vi "UHR-Fleezers Control (host) - 10.8MV_trial2.vi"() -> ()   [LabVIEW 2010] (continued)
        n272 = local read "Location path"() -> (w931:path)
        n273 = Reshape Array(w934, 12) -> (w932:string[])
        n274 = Write to Text File(file (use dialog)=w931, text=w932) -> ()  [unwired: 2 in, 3 out]
      }
      event "Activate Joystick": Value Change {
        n275 = event-data() -> ()  [unwired: 1 in, 5 out]
        n276 = case shown="True" "Activate Joystick" {
          frame False {
          }
          frame True {
            # "Change the trajectory mode to Jog"
            n277 = local read "ESP Port"() -> (w939:refnum<visa-resource-name>)
            n278 = Concatenate Strings("1TJ3;\n2TJ3;\n3TJ3" ("Substring"), "\r") -> (w936:string)
            n279 = VISA Write(VISA resource name=w939, write buffer=w936) -> ()  [unwired: 1 in, 3 out]
          }
        }
      }
    }
  }
  n280 = disable-structure shown="Disabled" {
    disable-tunnel: w24 -> [w968 _]
    frame Disabled {
      w963 = T17 0 items=["Grayscale (U8)", "Grayscale (I16)", "Grayscale (SGL)", "Complex (CSG)", "RGB (U32)", "HSL (U32)", "RGB (U64)", "Grayscale (U16)"] ("Image Type")
      n281 = call <vilib>:"IMAQ Init.vi"("Interface Name"="img0") -> ("error out"=w965:errorcluster, "IMAQ Session Out"=w967:refnum<k11>)  [unwired: 9 in]
      n282 = call <vilib>:"IMAQ Grab Setup.vi"("error in (no error)"=w965, "IMAQ Session In"=w967) -> ("error out"=w961:errorcluster, "IMAQ Session Out"=w962:refnum<k11>)  [unwired: 8 in]
      n283 = call "IMAQ Create"("Image Name"="untitled", "Image Type"=w963) -> ("New Image"=w960:T2)  [unwired: 3 in, 1 out]
      n284 = call <vilib>:"Application Directory.vi"() -> ("Application Directory"=w947:path)
      n285 = Build Path(base path=w947, name or relative path="_trap_screen_positions") -> (appended path=w955:path)
      n286 = Open/Create/Replace File(file path (use dialog)=w955, operation (0:open)=T25."open or create", access (0:read/write)=enum16{"read/write", "read-only", "write-only"}."read/write") -> (refnum out=w957:refnum<file>)  [unwired: 3 in, 2 out]
      n287 = local read "Trap Sets"() -> (w949:u32)
      n288 = for "Load trap positions on video screen from file." {
        N: w949 -> [_]
        tunnel: [w975] -> w950
        tunnel: w957 -> [w974]
        tunnel: [w971] -> w946 mode=indexing
        w973 = 4
        n289 = for {
          N: w973 -> [_]
          tunnel: [w979] -> w975
          tunnel: w974 -> [w978]
          tunnel: w973 -> [w977]
          tunnel: [w976] -> w972 mode=indexing
          n290 = Read from Binary File(5:w977, 11:w978) -> (2:w976:i32, 3:w979:refnum<file>)  [unwired: 4 in, 2 out]
        }
        n291 = Array To Cluster(array=w972) -> (cluster=w971:T29)
      }
      n292 = node-c288() -> (w970:T26)  [unwired: 4 in]
      n293 = timed-loop "acquire video and stage position" {
        timing: w970 -> [_]
        timing-out: [_] -> w969
        tunnel: w962 -> [w998]
        tunnel: w961 -> [w997]
        tunnel: w960 -> [w996]
        tunnel: [w995] -> w942
        tunnel: [w992] -> w943
        tunnel: [w993] -> w941
        tunnel: w968 -> [_]
        shift-right: [w989] -> w959
        shift-left: w946 -> [w990]
        tunnel: w949 -> [w987]
        stop <- w994 stop-if-true
        n294 = node-c288() -> ()  [unwired: 1 in, 1 out]
        n295 = event shown="[2] \"Primary Video Display\": Mouse Down" {
          selector: _ -> [_ _ _ _]
          dyn-events: _ -> [_ _ _ _]
          timeout: 10 -> [_ _ _ _]
          tunnel: w998 -> [w1009 w1024 w1033 w1052]
          tunnel: w997 -> [w1008 w1026 w1031 w1054]
          tunnel: w996 -> [w1007 w1025 w1032 w1053]
          tunnel: [w1006 w1024 w1033 w1052] -> w995
          tunnel: [w999 w1028 FALSE FALSE] -> w994
          tunnel: [w1003 w1026 w1031 w1054] -> w993
          tunnel: [w1002 w1025 w1032 w1053] -> w992
          tunnel: "radius" -> [_ _ w1038 _]
          tunnel: w990 -> [w1000 w1027 w1036 _]
          tunnel: [w1000 w1027 w1037 cluster{i32, i32, i32, i32}[] []] -> w989
          tunnel: w987 -> [_ _ w1029 _]
          event Timeout {
            n296 = event-data() -> ()  [unwired: 1 in, 2 out]
            n297 = call <vilib>:"IMAQ Grab Acquire.vi"("error in (no error)"=w1008, "Image In"=w1007, "IMAQ Session In"=w1009) -> ("error out"=w1004:errorcluster, "Image Out"=w1005:T2, "IMAQ Session Out"=w1006:refnum<k11>)  [unwired: 5 in, 1 out]
            n298 = case shown="True" "trap\nmarkers?" {
              tunnel: w1000 -> [_ w1017]
              tunnel: w1005 -> [w1011 w1016]
              tunnel: w1004 -> [w1010 w1015]
              tunnel: [w1010 w1014] -> w1003
              tunnel: [w1011 w1012] -> w1002
              frame False {
              }
              frame True {
                n299 = for {
                  tunnel: w1017 -> [w1023] mode=indexing
                  shift-right: [w1021] -> w1012
                  shift-left: w1016 -> [w1022]
                  tunnel: w1015 -> [w1020]
                  tunnel: [w1019] -> w1014
                  tunnel: u32 16711680 ("Color") -> [w1018]
                  n300 = call "IMAQ Overlay Oval"("Color"=w1018, "error in (no error)"=w1020, "Bounding Rectangle"=w1023, "Image"=w1022) -> ("error out"=w1019:errorcluster, "Image Out"=w1021:T2)  [unwired: 6 in]
                }
              }
            }
            "Primary Video Display" <- w1002
            n301 = Unbundle By Name(w1004) -> ("status"=w999:bool)
          }
          event "Stop All": Value Change {
            n302 = event-data() -> ()  [unwired: 1 in, 5 out]
            n303 = local read "Stop All"() -> (w1028:bool)
          }
          event "Primary Video Display": Mouse Down {
            n304 = event-data() -> ()  [unwired: 1 in, 7 out]
            n305 = Array Size(array=w1036) -> (size(s)=w1035:i32)
            n306 = Less?(x=w1035, y=w1029) -> (x < y?=w1034:bool)
            n307 = case shown="True" w1034 {
              tunnel: w1038 -> [_ w1048]
              tunnel: w1036 -> [w1039 w1042]
              tunnel: [w1039 w1041] -> w1037
              frame False {
              }
              frame True {
                n308 = property on="Primary Video Display" class="ImageControl"() -> ("Last Mouse Position"=w1040:cluster{"X":i32, "Y":i32})  [unwired: 2 in, 2 out]
                n309 = Unbundle By Name(w1040) -> ("X"=w1050:i32, "Y"=w1049:i32)
                n310 = Add(x=w1049, y=w1048) -> (x+y=w1046:i32)
                n311 = Subtract(x=w1049, y=w1048) -> (x-y=w1044:i32)
                n312 = Add(x=w1050, y=w1048) -> (x+y=w1045:i32)
                n313 = Subtract(x=w1050, y=w1048) -> (x-y=w1047:i32)
                n314 = Bundle(w1047, w1046, w1045, w1044) -> (w1043:cluster{i32, i32, i32, i32})  [unwired: 1 in]
                n315 = Build Array (concatenate)(w1042, w1043) -> (w1041:T30)
              }
            }
          }
          event "clear markers": Value Change {
            n316 = event-data() -> ()  [unwired: 1 in, 5 out]
          }
        }
        n317 = node-c288() -> ()  [unwired: 1 in, 1 out]
      }
      n318 = node-c288(w969) -> ()  [unwired: 1 out]
      n319 = Set File Position(offset (in bytes) (0)=i64 0, refnum=w950, from (0:start)=enum16{"start", "end", "current"}."start") -> (refnum out=w951:refnum<file>)  [unwired: 1 in, 1 out]
      n320 = for "Write trap positions to file so they can be remembered\nwhen program is removed from memory" {
        tunnel: w959 -> [w983] mode=indexing
        tunnel: [w981] -> w958
        tunnel: w951 -> [w980]
        n321 = Cluster To Array(cluster=w983) -> (array=w982:i32[])
        n322 = for {
          tunnel: w982 -> [w986] mode=indexing
          tunnel: [w985] -> w981
          tunnel: w980 -> [w984]
          n323 = Write to Binary File(file (use dialog)=w984, data=w986) -> (refnum out=w985:refnum<file>)  [unwired: 4 in, 2 out]
        }
      }
      n324 = Close File(refnum=w958) -> ()  [unwired: 1 in, 2 out]
      n325 = call "IMAQ Dispose"("Image"=w943, "error in (no error)"=w941) -> ("error out"=w940:errorcluster)  [unwired: 4 in]
      n326 = call <vilib>:"IMAQ Stop.vi"("error in (no error)"=w940, "IMAQ Session In"=w942) -> ("error out"=w944:errorcluster, "IMAQ Session Out"=w945:refnum<k11>)  [unwired: 8 in]
      n327 = call <vilib>:"IMAQ Close.vi"("error in (no error)"=w944, "IMAQ Session In"=w945) -> ()  [unwired: 9 in, 1 out]
    }
    frame Enabled {
    }
  }
  n328 = node-c288(2 ("Processor")) -> (w15:T26)  [unwired: 3 in]
  n329 = node-c288() -> (w69:T26)  [unwired: 4 in]
  n330 = disable-structure shown="Enabled" {
    disable-tunnel: [w1061 _] -> w35
    disable-tunnel: w24 -> [w1060 _]
    frame Enabled {
      n331 = node-c288() -> (w1063:T26)  [unwired: 4 out]
      n332 = timed-loop "Rough control of MCL mirror stage (debugging)" {
        tunnel: w1060 -> [w1066]
        tunnel: [w1065] -> w1061
        timing: w1063 -> [_]
        timing-out: [_] -> w1062
        stop <- w1065 stop-if-true
        n333 = node-c288() -> ()  [unwired: 2 out]
        n334 = case shown="1" "MCL Mode" {
          tunnel: w1066 -> [_ w1069 w1173]
          frame 0, Default {
            # "manual positioning"
          }
          frame 1 {
            # "sinusoidal wave"
            n335 = node-c288() -> (w1071:T26)  [unwired: 4 out]
            n336 = timed-loop "Oscillate MCL mirror" {
              timing: w1071 -> [_]
              timing-out: [_] -> w1070
              tunnel: w1069 -> [w1110]
              i -> [w1109]
              stop <- w1072 stop-if-true
              n337 = node-c288() -> (w1108:i64)  [unwired: 1 out]
              n338 = Multiply(x="AO1", y=32767.0) -> (x*y=w1104:dbl)
              n339 = Multiply(x="AO2", y=32767.0) -> (x*y=w1099:dbl)
              n340 = Divide(x=w1104, y=10.0) -> (x/y=w1105:dbl)
              n341 = Divide(x=w1099, y=10.0) -> (x/y=w1100:dbl)
              n342 = To Word Integer(number=w1105) -> (16bit integer=w1097:i16)
              n343 = To Word Integer(number=w1100) -> (16bit integer=w1096:i16)
              n344 = Divide(x=w1108, y=i64 1000) -> (x/y=w1079:dbl)
              n345 = Multiply(x=w1079, y=w1109) -> (x*y=w1090:dbl)
              n346 = Multiply(x="Osc. freq. (Hz) 2", y=6.283185307179586) -> (x*y=w1091:dbl)
              n347 = Multiply(x=w1091, y=w1090) -> (x*y=w1089:dbl)
              n348 = Sine(x=w1089) -> (sin(x)=w1088:dbl)
              n349 = Multiply(x=w1088, y="Osc. amp. (V)") -> (x*y=w1086:dbl)
              n350 = Add(x=w1086, y="Osc. center (V)") -> (x+y=w1084:dbl)
              n351 = Divide(x=w1084, y=10.0) -> (x/y=w1082:dbl)
              n352 = Multiply(x=w1082, y=32767.0) -> (x*y=w1077:dbl)
              n353 = Select(t=w1077, s="Scan axis", f=w1097) -> (s? t:f=w1095:dbl)
              n354 = Select(t=w1096, s="Scan axis", f=w1077) -> (s? t:f=w1094:dbl)
              n355 = local read "MCL Mode"() -> (w1076:u16)
              n356 = Not Equal?(x=w1076, y=u16 1) -> (x != y?=w1073:bool)
              n357 = local read "Stop All"() -> (w1074:bool)
              n358 = xnode "Read/Write Control"("FPGA VI Reference In"=w1110, "AO1"=w1095, "AO2"=w1094) -> ()  [unwired: 1 in, 2 out]
              n359 = Compound Arithmetic op=OR(w1074, w1073) -> (w1072:bool)
              n360 = node-c288() -> ()  [unwired: 2 out]
            }
            n361 = node-c288(w1070) -> ()  [unwired: 1 out]
          }
          frame 2 {
            # "linear scan"
            n362 = case shown="True" "Start Scan" {
              tunnel: w1173 -> [_ w1185]
              frame False {
              }
              frame True {
                n363 = Subtract(x="End (V)", y="Begin (V)") -> (x-y=w1181:dbl)
                n364 = Decrement(x="N Points") -> (x-1=w1180:dbl)
                n365 = Divide(x=w1181, y=w1180) -> (x/y=w1178:dbl)
                n366 = for {
                  N: "N Points" -> [_]
                  tunnel: "Begin (V)" -> [w1198]
                  tunnel: w1185 -> [w1190]
                  tunnel: [w1189] -> w1184 mode=indexing
                  tunnel: w1178 -> [w1188]
                  tunnel: [w1186] -> w1177 mode=indexing
                  i -> [w1197]
                  n367 = Multiply(x=w1188, y=w1197) -> (x*y=w1196:dbl)
                  n368 = Add(x=w1198, y=w1196) -> (x+y=w1193:dbl)
                  n369 = local read "Scan axis"() -> (w1187:bool)
                  n370 = local read "AO1"() -> (w1195:dbl)
                  n371 = local read "AO2"() -> (w1194:dbl)
                  n372 = Select(t=w1193, s=w1187, f=w1195) -> (s? t:f=w1192:dbl)
                  n373 = Select(t=w1194, s=w1187, f=w1193) -> (s? t:f=w1191:dbl)
                  n374 = flat-sequence {
                    tunnel: w1192 -> [w1202]
                    tunnel: w1191 -> [w1201]
                    tunnel: w1190 -> [w1199]
                    tunnel: [w1269] -> w1189
                    tunnel: [w1268] -> w1186
                    frame #0 {
                      w1205 = 10.0 ("y")
                      w1200 = 32767.0 ("y")
                      n375 = Multiply(x=w1202, y=w1200) -> (x*y=w1208:dbl)
                      n376 = Multiply(x=w1201, y=w1200) -> (x*y=w1206:dbl)
                      n377 = Divide(x=w1208, y=w1205) -> (x/y=w1209:dbl)
                      n378 = Divide(x=w1206, y=w1205) -> (x/y=w1207:dbl)
                      n379 = To Word Integer(number=w1209) -> (16bit integer=w1203:i16)
                      n380 = To Word Integer(number=w1207) -> (16bit integer=w1204:i16)
                      n381 = xnode "Read/Write Control"("FPGA VI Reference In"=w1199, "AO1"=w1203, "AO2"=w1204) -> ()  [unwired: 1 in, 2 out]
                    }
                    frame #1 {
                      n382 = Wait (ms)(milliseconds to wait="DAQ Delay (ms)") -> ()  [unwired: 1 out]
                    }
                    frame #2 {
                      n383 = local read "Slow mean"() -> (w1269:dbl)
                      n384 = local read "Sigma"() -> (w1268:dbl)
                    }
                  }
                }
                n385 = Bundle("Begin (V)"="Begin (V)", w1178, w1184) -> (→"MCL Scan":cluster{"Begin (V)":dbl, dbl, dbl[]})  [unwired: 1 out]
                n386 = Bundle("Begin (V)"="Begin (V)", w1178, w1177) -> (→"MCL Scan 2":cluster{"Begin (V)":dbl, dbl, dbl[]})  [unwired: 1 out]
              }
            }
          }
        }
        n387 = local read "Stop All"() -> (w1065:bool)
        n388 = node-c288() -> ()  [unwired: 2 out]
      }
      n389 = node-c288(w1062) -> ()  [unwired: 1 out]
    }
    frame Disabled {
    }
  }
  n390 = timed-loop "Control parameters (event loop)" {
    tunnel: w24 -> [w1275]
    shift-right: [w1274] -> _
    shift-left: errorcluster {"status"=FALSE, "code"=0, "source"=""} ("error out") -> [w1273]
    tunnel: [w1272] -> w37
    timing: w15 -> [_]
    timing-out: [_] -> w14
    stop <- w1272 stop-if-true
    n391 = node-c288() -> ()  [unwired: 1 in, 1 out]
    n392 = event shown="[6] \"BD 1 Frequency 1 (MHz)\", \"BD 1 Frequency 2 (MHz)\", \"BD 1 Frequency 3 (MHz)\", \"BD 2 Frequency 1 (MHz)\", \"BD 2 Frequency 2 (MHz)\", \"BD 2 Frequency 3 (MHz)\", \"Trap Delta (MHz)\": Value Change" {
      selector: _ -> [_ _ _ _ _ _ _ _ _ _ _ _ _ _ _ _ _ _ _ _ _ _ _ _ _ _ _ _ _ _ _ _ _ _ _ _ _ _ _ _ _ _ _ _ _ _ _ _ _ _ _ _ _ _ _]
      dyn-events: _ -> [_ _ _ _ _ _ _ _ _ _ _ _ _ _ _ _ _ _ _ _ _ _ _ _ _ _ _ _ _ _ _ _ _ _ _ _ _ _ _ _ _ _ _ _ _ _ _ _ _ _ _ _ _ _ _]
      timeout: _ -> [_ _ _ _ _ _ _ _ _ _ _ _ _ _ _ _ _ _ _ _ _ _ _ _ _ _ _ _ _ _ _ _ _ _ _ _ _ _ _ _ _ _ _ _ _ _ _ _ _ _ _ _ _ _ _]
      tunnel: w1275 -> [w1313 _ _ _ w1435 _ w1532 _ w1596 _ _ _ w1791 _ _ w1893 w2037 w2101 w2176 w2330 w2407 w2538 w2634 w2720 w2806 w2892 w2978 w3064 w3157 w3321 w3532 _ w3677 w3814 _ w4021 w4063 w4111 w4190 w4232 _ w4278 _ _ _ _ w4469 _ w4562 w4603 w4650 w4838 w4887 _ w4949]
      tunnel: [w1312 _ _ _ w1425 _ w1531 _ w1559 _ w1756 _ w1770 _ _ w1892 w2033 w2098 w2173 w2329 w2405 w2537 w2628 w2714 w2800 w2886 w2972 w3058 w3155 w3320 w3530 _ w3675 w3812 _ w4019 w4061 w4101 w4188 w4230 _ w4276 _ _ _ _ w4467 _ _ _ _ _ _ _ _] -> w1274
      tunnel: w1273 -> [w1311 _ _ _ w1434 _ w1530 _ w1591 _ w1756 _ w1790 _ _ w1891 w2032 w2097 w2172 w2328 w2406 w2536 w2633 w2719 w2805 w2891 w2977 w3063 w3156 w3319 w3531 _ w3676 w3813 _ w4020 w4062 w4110 w4189 w4231 _ w4277 _ _ _ _ w4468 _ w4561 w4602 w4649 w4837 w4886 _ w4948]
      tunnel: [_ _ _ _ _ _ _ _ _ _ w1755 _ _ _ _ _ _ _ _ _ _ _ _ _ _ _ _ _ _ _ _ _ _ _ _ _ _ _ _ _ _ _ _ _ _ _ _ _ _ _ _ _ _ _ _] -> w1272
      tunnel: [_ _ _ _ _ _ _ "Round T1 X" _ _ _ _ _ _ _ _ _ _ _ _ _ _ _ _ _ _ _ _ _ _ _ _ _ _ _ _ _ _ _ _ _ _ _ _ _ _ _ _ _ _ _ _ _ _ _] -> _
      tunnel: [_ _ _ "Adjust Scale\nto Mean" _ _ _ _ _ _ _ _ _ _ _ _ _ _ _ _ _ _ _ _ _ _ _ _ _ _ _ _ _ _ _ _ _ _ _ _ _ _ _ _ _ _ _ _ _ _ _ _ "Set SP to Reading" _ _] -> _
      tunnel: [_ _ _ _ _ _ _ _ _ "Round T2 X" _ "Delayed Interlace Start" _ _ _ _ _ _ _ _ _ _ _ _ _ _ _ _ _ _ _ _ _ _ _ _ _ _ _ _ _ _ _ _ _ _ _ _ _ _ _ _ _ _ _] -> _
      event "AI Count (ticks)", "Sets to FIFO (Traps)", "Save ave N", "FPGA Ave.", "# Samples/channel", "N sets to save": Value Change {
        # "So that if 'Save ave N' is updated, the AOD scanning code updates too."
        n393 = event-data() -> ()  [unwired: 6 out]
        n394 = local read "AI Count (ticks)"() -> (w1293:u32)
        n395 = Boolean To (0,1)(Boolean="Sets to FIFO (Traps)") -> (0, 1=w1303:cluster{"Set 1":i16, "Set 2":i16, "Set 3":i16})
        n396 = xnode "Read/Write Control"("FPGA VI Reference In"=w1313, "error in"=w1311, "ai count"=w1293, "AI1 Sets to FIFO"="Sets to FIFO (Traps)", "N of AI1 Int Acq Sets"="N Acq Sets (Traps + Fl.)") -> ("error out"=w1312:errorcluster)  [unwired: 1 out]
        n397 = Cluster To Array(cluster=w1303) -> (array=w1302:i16[])
        n398 = To Unsigned Long Integer(number=w1302) -> (unsigned 32bit integer=w1282:u32[])
        n399 = local read "Scan steps (AOD)"() -> (w1304:u64)
        n400 = Multiply(x=w1293, y="N Acq Sets (Traps + Fl.)") -> (x*y=w1291:u32)
        n401 = Divide(x=40000000.0, y=w1293) -> (x/y=w1285:dbl)
        "AI rate (Hz)" <- w1285
        "Ave. Rate (Hz)" <- w1285
        n402 = Add Array Elements(numeric array=w1282) -> (sum=w1294:u32)
        "Trap Sets" <- w1294
        n403 = Reciprocal(x=w1285) -> (1/x=→"Ave. Period (s)":dbl)
        n404 = property on="Scan steps (AOD)" class="DigNum (strict)"("Val(Sgnl)"=w1304) -> ()  [unwired: 2 in, 2 out]
        n405 = Divide(x=w1285, y="N Acq Sets (Traps + Fl.)") -> (x/y=w1308:dbl)
        "Data Rate (Hz)" <- w1308
        n406 = Reciprocal(x=w1308) -> (1/x=→"Data Period (s)":dbl)
        n407 = local read "Save ave N"() -> (w1307:dbl)
        n408 = Divide(x=w1308, y=w1307) -> (x/y=w1306:dbl)
        "Save Data Rate (Hz)" <- w1306
        n409 = Reciprocal(x=w1306) -> (1/x=→"Save Data Period (s)":dbl)
        n410 = Multiply(x=w1291, y="# Samples/trap") -> (x*y=w1289:u32)
        "Counts/DMA" <- w1289
        n411 = property on="Trap Disp. Downsample" class="DigNum (strict)"("Maximum"="# Samples/trap") -> ()  [unwired: 2 in, 2 out]
        n412 = Multiply(x=w1294, y="# Samples/trap") -> (x*y=w1283:u32)
        "# Samples/channel" <- w1283
        n413 = Multiply(x=w1283, y=u32 8) -> (x*y=→"Trap AI Elements/DMA read":u32)
        n414 = local read "APD Int. Count"() -> (w1290:u32)
        n415 = Multiply(x=w1283, y=u32 3) -> (x*y=→"Trap Pos Elements/DMA read":u32)
        n416 = Divide(x=w1289, y=w1290) -> (x/y=w1280:dbl)
        "APD Samples/FIFO Acq." <- w1280
        n417 = Divide(x=w1289, y=40000000.0) -> (x/y=w1287:dbl)
        "DMA Update Period (s)" <- w1287
        n418 = Multiply(x=2.0, y=w1280) -> (x*y=→"APD Elements/DMA read":dbl)
        n419 = property on="APD Disp. Downsample" class="DigNum (strict)"("Maximum"=w1280) -> ()  [unwired: 2 in, 2 out]
        n420 = local read "N sets to save"() -> (w1300:u32)
        n421 = Multiply(x=w1287, y=w1300) -> (x*y=→"Total Time (s)":dbl)
        "FPGA Averaging" <- FALSE ("FPGA Averaging")
      }
      event "Rescale on Mean": Value Change {
        n422 = event-data() -> ()  [unwired: 7 out]
        n423 = And(x=FALSE, y="Rescale on Mean") -> (x .and. y?=w1400:bool)
        n424 = local write "Rescale on Mean"(w1400) -> ()
        n425 = local read "Bead Mean (nm)"() -> (w1405:dbl)
        n426 = Add(x="Amplitude (nm)", y=w1405) -> (x+y=w1403:dbl)
        n427 = Subtract(x=w1405, y="Amplitude (nm)") -> (x-y=w1402:dbl)
        n428 = property on="Bead Separation" class="WFChart (strict)"("YScale.Minimum"=w1402) -> ()  [unwired: 2 in, 2 out]
        n429 = property on="Bead Separation" class="WFChart (strict)"("YScale.Maximum"=w1403) -> ()  [unwired: 2 in, 2 out]
      }
      event "Detector Type": Value Change {
        n430 = event-data() -> ()  [unwired: 7 out]
        n431 = local read "AI labels"() -> (w1406:string[])
        n432 = property on="High Res. Display" class="Ring (strict)"("Strings []"=w1406) -> ()  [unwired: 2 in, 2 out]
        n433 = Build Array (concatenate)(w1406, "none") -> (w1407:string[])
        n434 = property on="FFT 1 Choice 1" class="Ring (strict)"("Strings []"=w1407) -> ()  [unwired: 2 in, 2 out]
        n435 = property on="FFT 1 Choice 2" class="Ring (strict)"("Strings []"=w1407) -> ()  [unwired: 2 in, 2 out]
        n436 = property on="FFT 2 Choice 1" class="Ring (strict)"("Strings []"=w1407) -> ()  [unwired: 2 in, 2 out]
        n437 = property on="FFT 2 Choice 2" class="Ring (strict)"("Strings []"=w1407) -> ()  [unwired: 2 in, 2 out]
        n438 = Bundle("APD 1", "APD 2") -> (w1410:cluster{string, string})  [unwired: 1 out]
        n439 = Cluster To Array(cluster=w1410) -> (array=w1408:string[])
        n440 = Build Array (concatenate)(w1408, w1407) -> (w1412:string[])
        n441 = Array Size(array=w1412) -> (size(s)=w1413:i32)
        n442 = property on="Signals to Plot" class="LstBox (strict)"("Item Names"=w1412) -> ()  [unwired: 2 in, 2 out]
        n443 = property on="Signals to Plot" class="LstBox (strict)"("Number of Rows"=w1413) -> ()  [unwired: 2 in, 2 out]
        n444 = property on="All Signals" class="WFChart (strict)"("LegNumRows"=w1413) -> ()  [unwired: 2 in, 2 out]
      }
      event "Adjust Scale\nto Mean": Value Change {
        n445 = event-data() -> ()  [unwired: 7 out]
        n446 = local read "APD 1 Rate (Hz)"() -> (w1422:dbl)
        n447 = Multiply(x=1000.0, y="Above (kHz)") -> (x*y=w1420:dbl)
        n448 = Multiply(x=1000.0, y="Below (kHz)") -> (x*y=w1418:dbl)
        n449 = Add(x=w1420, y=w1422) -> (x+y=w1415:dbl)
        n450 = Subtract(x=w1422, y=w1418) -> (x-y=w1416:dbl)
        n451 = property on="APD Chart" class="WFChart (strict)"("YScale.Minimum"=w1416) -> ()  [unwired: 2 in, 2 out]
        n452 = property on="APD Chart" class="WFChart (strict)"("YScale.Maximum"=w1415) -> ()  [unwired: 2 in, 2 out]
      }
      event "Phase adj. (AI1)", "+ phase (AI1)", "- phase (AI1)": Value Change {
        n453 = event-data() -> ()  [unwired: 7 out]
        n454 = Negate(x="Phase adj. (AI1)") -> (-x=w1432:i16)
        n455 = Select(t=w1432, s="- phase (AI1)", f="Phase adj. (AI1)") -> (s? t:f=w1431:i16)
        n456 = xnode "Read/Write Control"("FPGA VI Reference In"=w1435, "error in"=w1434, "Phase count adjustment"=w1431) -> ("FPGA VI Reference Out"=w1430:T19, "error out"=w1429:errorcluster)
        n457 = Or(x="- phase (AI1)", y="+ phase (AI1)") -> (x .or. y?=w1426:bool)
        n458 = xnode "Read/Write Control"("FPGA VI Reference In"=w1430, "error in"=w1429, "+ phase"=w1426) -> ("error out"=w1425:errorcluster)  [unwired: 1 out]
      }
      event "Signals to Plot": Double Click {
        w1513 = u32 9868950 ("Color Box")
        n459 = event-data() -> ("Row"=w1515:i32)  [unwired: 9 out]
        n460 = property on="All Signals" class="WFChart (strict)"("Active Plot"=w1515) -> (error out=w1526:errorcluster)  [unwired: 2 in, 1 out]
        n461 = property on="All Signals" class="WFChart (strict)" props=["Plot", "Visible?", "Plot", "Plot Color"](error in=w1526) -> (error out=w1525:errorcluster, "Plot.Visible?"=w1524:bool)  [unwired: 1 in, 2 out]
        n462 = Select(t=FALSE ("Plot.Visible"), s=w1524, f=TRUE ("Plot.Visible")) -> (s? t:f=w1519:bool)
        n463 = property on="All Signals" class="WFChart (strict)"(error in=w1525, "Plot.Visible?"=w1519) -> (error out=w1521:errorcluster)  [unwired: 1 in, 1 out]
        n464 = property on="All Signals" class="WFChart (strict)"(error in=w1521) -> (error out=w1516:errorcluster, "Plot.Plot Color"=w1520:u32)  [unwired: 1 in, 1 out]
        n465 = property on="Signals to Plot" class="LstBox (strict)"(error in=w1516, "Active Row"=w1515) -> (error out=w1514:errorcluster)  [unwired: 1 in, 1 out]
        n466 = Select(t=w1520, s=w1519, f=u32 0) -> (s? t:f=w1517:u32)
        n467 = property on="Signals to Plot" class="LstBox (strict)"(error in=w1514, "CellFontColor"=w1517, "SelColor"=w1513, "CellBG"=w1513, "CellFontSize"=u32 20 ("Active Row:Cell Font:Size"), "CellFontBold"=TRUE ("Active Row:Cell Font:Bold")) -> ()  [unwired: 1 in, 2 out]
      }
      event "BD 1 Frequency 1 (MHz)", "BD 1 Frequency 2 (MHz)", "BD 1 Frequency 3 (MHz)", "BD 2 Frequency 1 (MHz)", "BD 2 Frequency 2 (MHz)", "BD 2 Frequency 3 (MHz)", "Trap Delta (MHz)": Value Change {
        # "anytime one of the frequencies is changed, write it to the RF board UNLESS Set 2 is being oscillated. The oscillation\nscript writes the frequencies to the RF board."
        n468 = event-data() -> ("CtlRef"=w1529:refnum<vi>)  [unwired: 6 out]
        n469 = control-ref of="Trap Delta (MHz)"() -> (w1528:refnum<vi>)
        n470 = Equal?(x=w1528, y=w1529) -> (x = y?=w1527:bool)
        n471 = case shown="False" "Oscillate Set 2" {
          tunnel: w1532 -> [w1552 _]
          tunnel: [w1551 w1555] -> w1531
          tunnel: w1530 -> [w1550 w1555]
          tunnel: w1527 -> [w1536 _]
          frame False {
            n472 = local read "BD 1 Frequency 1 (MHz)"() -> (w1534:dbl)
            n473 = local read "BD 1 Frequency 2 (MHz)"() -> (w1538:dbl)
            n474 = Add(x=w1534, y="Trap Delta (MHz)") -> (x+y=w1537:dbl)
            n475 = Select(t=w1537, s=w1536, f=w1538) -> (s? t:f=w1535:dbl)
            n476 = local read "Y RF Frequency Limits (MHz)"() -> (w1540:T16)
            n477 = local read "X RF Frequency Limits (MHz)"() -> (w1541:T16)
            n478 = local read "BD 1 Frequency 3 (MHz)"() -> (w1553:dbl)
            n479 = local write "BD 1 Frequency 2 (MHz)"(w1535) -> ()
            n480 = local read "BD 2 Frequency 1 (MHz)"() -> (w1544:dbl)
            n481 = local read "BD 2 Frequency 2 (MHz)"() -> (w1543:dbl)
            n482 = local read "BD 2 Frequency 3 (MHz)"() -> (w1554:dbl)
            n483 = call "set RF board frequency - interlace.vi"("Board 2 Frequency Limits"=w1540, "Board 1 Frequency Limits"=w1541, "error in"=w1550, "FPGA VI Reference In"=w1552, "Board 2 Frequency 3 (MHz)"=w1554, "Board 1 Frequency 3 (MHz)"=w1553, "Board 2 Frequency 2 (MHz)"=w1543, "Board 2 Frequency 1 (MHz)"=w1544, "Board 1 Frequency 2 (MHz)"=w1535, "Board 1 Frequency 1  (MHz)"=w1534) -> ("error out"=w1551:errorcluster)  [unwired: 1 out]
            n484 = Subtract(x=w1544, y=w1543) -> (x-y=w1548:dbl)
            n485 = Subtract(x=w1535, y=w1534) -> (x-y=w1549:dbl)
            n486 = Square(x=w1548) -> (x^2=w1546:dbl)
            n487 = Square(x=w1549) -> (x^2=w1547:dbl)
            n488 = Add(x=w1547, y=w1546) -> (x+y=w1545:dbl)
            n489 = Square Root(x=w1545) -> (sqrt(x)=w1542:dbl)
            n490 = local write "Trap Delta (MHz)"(w1542) -> ()
            n491 = property on="Initial delta (MHz)" class="DigNum (strict)"("Val(Sgnl)"=w1542) -> ()  [unwired: 2 in, 2 out]
          }
          frame True {
          }
        }
      }
      event "Round T1 X": Value Change {
        n492 = event-data() -> ()  [unwired: 7 out]
        n493 = local read "BD 1 Frequency 1 (MHz)"() -> (w1558:dbl)
        n494 = Round To Nearest(number=w1558) -> (nearest integer value=w1557:dbl)
        n495 = property on="BD 1 Frequency 1 (MHz)" class="DigNum (strict)"("Val(Sgnl)"=w1557) -> ()  [unwired: 2 in, 2 out]
      }
      event "Restart RF": Value Change {
        n496 = event-data() -> ()  [unwired: 7 out]
        n497 = xnode "Read/Write Control"("FPGA VI Reference In"=w1596, "error in"=w1591, "FPGA Controls  RF Box"=FALSE) -> ("FPGA VI Reference Out"=w1595:T19, "error out"=w1590:errorcluster)
        n498 = local read "Y RF Amplitude Limits (%)"() -> (w1571:T16)
        n499 = local read "X RF Amplitude Limits (%)"() -> (w1572:T16)
        n500 = local read "X RF Frequency Limits (MHz)"() -> (w1574:T16)
        n501 = local read "Y RF Frequency Limits (MHz)"() -> (w1573:T16)
        n502 = xnode "Read/Write Control"("FPGA VI Reference In"=w1595, "error in"=w1590, "Direct RF Box  Communication"=TRUE) -> ("FPGA VI Reference Out"=w1594:T19, "error out"=w1589:errorcluster)
        n503 = local read "BD 2 Frequency 3 (MHz)"() -> (w1581:dbl)
        n504 = local read "BD 2 Frequency 2 (MHz)"() -> (w1582:dbl)
        n505 = local read "BD 1 Frequency 3 (MHz)"() -> (w1585:dbl)
        n506 = local read "BD 1 Frequency 1 (MHz)"() -> (w1586:dbl)
        n507 = local read "BD 2 Frequency 1 (MHz)"() -> (w1583:dbl)
        n508 = local read "BD 1 Frequency 2 (MHz)"() -> (w1584:dbl)
        n509 = call "Initialize RF boards - interlace 3.vi"("error in"=w1589, "FPGA VI Reference In"=w1594) -> ("error out"=w1588:errorcluster, "FPGA VI Reference Out"=w1593:T19)
        n510 = local read "BD 2 Amplitude 2 (%)"() -> (w1576:dbl)
        n511 = local read "BD 2 Amplitude 1 (%)"() -> (w1577:dbl)
        n512 = local read "BD 2 Amplitude 3 (%)"() -> (w1575:dbl)
        n513 = local read "BD 1 Amplitude 3 (%)"() -> (w1580:dbl)
        n514 = local read "BD 1 Amplitude 1 (%)"() -> (w1579:dbl)
        n515 = local read "BD 1 Amplitude 2 (%)"() -> (w1578:dbl)
        n516 = call "set RF board frequency - interlace.vi"("Board 2 Frequency Limits"=w1573, "Board 1 Frequency Limits"=w1574, "error in"=w1588, "FPGA VI Reference In"=w1593, "Board 2 Frequency 3 (MHz)"=w1581, "Board 1 Frequency 3 (MHz)"=w1585, "Board 2 Frequency 2 (MHz)"=w1582, "Board 2 Frequency 1 (MHz)"=w1583, "Board 1 Frequency 2 (MHz)"=w1584, "Board 1 Frequency 1  (MHz)"=w1586) -> ("error out"=w1587:errorcluster, "FPGA VI Reference Out"=w1592:T19)
        n517 = call "set RF board amplitude - interlace.vi"("Board 2 Amplitude Limits"=w1571, "Board 1 Amplitude Limits"=w1572, "error in"=w1587, "FPGA VI Reference In"=w1592, "Board 2 Amplitude 3 (%)"=w1575, "Board 1 Amplitude 3 (%)"=w1580, "Board 2 Amplitude 2 (%)"=w1576, "Board 2 Amplitude 1 (%)"=w1577, "Board 1 Amplitude 2 (%)"=w1578, "Board 1 Amplitude 1 (%)"=w1579) -> ("error out"=w1564:errorcluster, "FPGA VI Reference Out"=w1568:T19)
        n518 = xnode "Read/Write Control"("FPGA VI Reference In"=w1568, "error in"=w1564, "Direct RF Box  Communication"=FALSE) -> ("FPGA VI Reference Out"=w1567:T19, "error out"=w1566:errorcluster)
        n519 = flat-sequence {
          tunnel: w1566 -> [w1597]
          tunnel: [w1597] -> w1565
          frame #0 {
            n520 = Wait (ms)(milliseconds to wait=u32 50) -> ()  [unwired: 1 out]
          }
        }
        n521 = xnode "Read/Write Control"("FPGA VI Reference In"=w1567, "error in"=w1565, "FPGA Controls  RF Box"=TRUE) -> ("error out"=w1560:errorcluster)  [unwired: 1 out]
        n522 = property on="Restart RF" class="Bool (strict)"(error in=w1560, "Value"=FALSE ("Restart RF")) -> (error out=w1559:errorcluster)  [unwired: 1 in, 1 out]
      }
      event "Round T2 X": Value Change {
        n523 = event-data() -> ()  [unwired: 7 out]
        n524 = local read "BD 1 Frequency 2 (MHz)"() -> (w1752:dbl)
        n525 = Round To Nearest(number=w1752) -> (nearest integer value=w1751:dbl)
        n526 = property on="BD 1 Frequency 2 (MHz)" class="DigNum (strict)"("Val(Sgnl)"=w1751) -> ()  [unwired: 2 in, 2 out]
      }
      event "Stop All": Value Change {
        n527 = event-data() -> ()  [unwired: 7 out]
        n528 = call "hamilton_controller.vi"("action"=T22."DISCONNECT") -> ()  [unwired: 10 in, 1 out]
        n529 = local read "Stop All"() -> (w1755:bool)
      }
      event "Delayed Interlace Start": Value Change {
        n530 = event-data() -> ()  [unwired: 7 out]
        n531 = flat-sequence {
          frame #0 {
            n532 = Multiply(x="Delay to Interlace (s)", y=1000.0) -> (x*y=w1758:dbl)
            n533 = Wait (ms)(milliseconds to wait=w1758) -> ()  [unwired: 1 out]
          }
          frame #1 {
            n534 = property on="Green laser mode" class="RadioBtnsControl (strict)"("Val(Sgnl)"=enum32{"Laser ON", "Laser OFF", "Interlace"}."Interlace" ("Value (Signaling)")) -> ()  [unwired: 2 in, 2 out]
          }
        }
      }
      event "BD 1 Amplitude 1 (%)", "BD 1 Amplitude 2 (%)", "BD 1 Amplitude 3 (%)", "BD 2 Amplitude 1 (%)", "BD 2 Amplitude 2 (%)", "BD 2 Amplitude 3 (%)", "Trap 1 ON", "Trap 2 ON", "Trap 3 ON", "Feedback On/Off", "All FB On/Off": Value Change {
        w1782 = i16 1 ("f")
        n535 = event-data() -> ()  [unwired: 7 out]
        n536 = local write "Trap 1 (ON/OFF)"("Trap 1 ON") -> ()
        n537 = local write "Trap 2 (ON/OFF)"("Trap 2 ON") -> ()
        n538 = Boolean To (0,1)(Boolean="Trap 3 ON") -> (0, 1=w1783:i16)
        n539 = Boolean To (0,1)(Boolean="Trap 1 ON") -> (0, 1=w1784:i16)
        n540 = Boolean To (0,1)(Boolean="Trap 2 ON") -> (0, 1=w1785:i16)
        n541 = Select(t=w1785, s="Trap ON/OFF X or Y Amp?", f=w1782) -> (s? t:f=w1780:i16)
        n542 = Select(t=w1784, s="Trap ON/OFF X or Y Amp?", f=w1782) -> (s? t:f=w1781:i16)
        n543 = Select(t=w1783, s="Trap ON/OFF X or Y Amp?", f=w1782) -> (s? t:f=w1779:i16)
        n544 = Select(t=w1782, s="Trap ON/OFF X or Y Amp?", f=w1785) -> (s? t:f=w1777:i16)
        n545 = Select(t=w1782, s="Trap ON/OFF X or Y Amp?", f=w1784) -> (s? t:f=w1778:i16)
        n546 = Select(t=w1782, s="Trap ON/OFF X or Y Amp?", f=w1783) -> (s? t:f=w1776:i16)
        n547 = And(x="All FB On/Off", y="Feedback On/Off") -> (x .and. y?=w1774:cluster{"Set 1":bool, "Set 2":bool})
        n548 = local read "BD 1 Amplitude 1 (%)"() -> (w1794:dbl)
        n549 = local read "BD 1 Amplitude 2 (%)"() -> (w1793:dbl)
        n550 = local read "BD 1 Amplitude 3 (%)"() -> (w1792:dbl)
        n551 = Unbundle By Name(w1774) -> ("Set 1"=w1769:bool, "Set 2"=w1766:bool)
        n552 = local read "Y RF Amplitude Limits (%)"() -> (w1762:T16)
        n553 = local read "X RF Amplitude Limits (%)"() -> (w1763:T16)
        n554 = local read "BD 2 Amplitude 1 (%)"() -> (w1795:dbl)
        n555 = local read "BD 2 Amplitude 2 (%)"() -> (w1796:dbl)
        n556 = local read "BD 2 Amplitude 3 (%)"() -> (w1797:dbl)
        n557 = And(x="Trap 2 ON", y=w1766) -> (x .and. y?=w1764:bool)
        n558 = And(x="Trap 1 ON", y=w1769) -> (x .and. y?=w1767:bool)
        n559 = Multiply(x=w1781, y=w1794) -> (x*y=w1789:dbl)
        n560 = Multiply(x=w1793, y=w1780) -> (x*y=w1787:dbl)
        n561 = Multiply(x=w1792, y=w1779) -> (x*y=w1788:dbl)
        n562 = Multiply(x=w1795, y=w1778) -> (x*y=w1798:dbl)
        n563 = Multiply(x=w1796, y=w1777) -> (x*y=w1799:dbl)
        n564 = Multiply(x=w1797, y=w1776) -> (x*y=w1800:dbl)
        n565 = call "set RF board amplitude - interlace.vi"("Board 2 Amplitude Limits"=w1762, "Board 1 Amplitude Limits"=w1763, "error in"=w1790, "FPGA VI Reference In"=w1791, "Board 2 Amplitude 3 (%)"=w1800, "Board 1 Amplitude 3 (%)"=w1788, "Board 2 Amplitude 2 (%)"=w1799, "Board 2 Amplitude 1 (%)"=w1798, "Board 1 Amplitude 2 (%)"=w1787, "Board 1 Amplitude 1 (%)"=w1789) -> ("error out"=w1771:errorcluster, "FPGA VI Reference Out"=w1772:T19)
        n566 = xnode "Read/Write Control"("FPGA VI Reference In"=w1772, "error in"=w1771, "FB On/Off Set 1"=w1767, "FB On/Off Set 2"=w1764) -> ("error out"=w1770:errorcluster)  [unwired: 1 out]
      }
      event "Load parameters": Value Change {
        n567 = event-data() -> ()  [unwired: 7 out]
        n568 = property on="Saved AOD Raster Scan Parameter Sets" class="Arr (strict)"() -> ("Index Values"=w1870:u32[])  [unwired: 2 in, 2 out]
        n569 = Index Array(array=w1870, index=0) -> (element=w1867:u32)
        n570 = local write "Load parameters"(FALSE ("Load parameters")) -> ()
        n571 = Index Array(array="Saved AOD Raster Scan Parameter Sets", index=w1867) -> (element=w1866:T32)
        n572 = Unbundle By Name(w1866) -> ("Scan Range AOD (nm) 2"=w1865:dbl, "Step Size AOD (nm) 2"=w1864:dbl, "Scan Speed AOD (nm/s) 2"=w1863:dbl, "Number of scans (AOD) 2"=w1862:u16)
        n573 = flat-sequence {
          tunnel: w1865 -> [w1873]
          tunnel: w1864 -> [w1872]
          tunnel: w1863 -> [w1871]
          tunnel: w1862 -> [w1874]
          frame #0 {
            n574 = local write "Scan Speed (nm/s)"(w1871) -> ()
            n575 = local write "Scan Range (nm)"(w1873) -> ()
            n576 = local write "Step Size (nm)"(w1872) -> ()
          }
          frame #1 {
            n577 = property on="Number of F/B Scans (AOD)" class="DigNum (strict)"("Val(Sgnl)"=w1874) -> ()  [unwired: 2 in, 2 out]
          }
        }
      }
      event "Trap 1 (ON/OFF)", "Trap 2 (ON/OFF)": Value Change {
        n578 = event-data() -> ()  [unwired: 7 out]
        n579 = property on="Trap 2 ON" class="Bool (strict)"("Val(Sgnl)"="Trap 2 (ON/OFF)") -> ()  [unwired: 2 in, 2 out]
        n580 = property on="Trap 1 ON" class="Bool (strict)"("Val(Sgnl)"="Trap 1 (ON/OFF)") -> ()  [unwired: 2 in, 2 out]
      }
      event "DIO count 1 (ticks)", "DIO count 2 (ticks)", "DIO count 3 (ticks)", "Interlace", "Number Interlace Sets", "Not-Interlacing Set": Value Change {
        n581 = event-data() -> ()  [unwired: 7 out]
        n582 = local read "DIO count 3 (ticks)"() -> (w1887:u32)
        n583 = local read "DIO count 1 (ticks)"() -> (w1889:u32)
        n584 = local read "DIO count 2 (ticks)"() -> (w1888:u32)
        n585 = To Unsigned Byte Integer(number="Not-Interlacing Set") -> (unsigned 8bit integer=w1878:u8)
        n586 = Add(x=w1878, y=u8 1) -> (x+y=w1882:u8)
        n587 = xnode "Read/Write Control"("FPGA VI Reference In"=w1893, "error in"=w1891, "DIO count 1 (ticks)"=w1889, "DIO count 2 (ticks)"=w1888, "DIO count 3 (ticks)"=w1887, "Interlace ON/OFF"="Interlace", "Number Interlace Cycles"="Number Interlace Sets", "Interlace Off Parameters"=w1882) -> ("error out"=w1892:errorcluster)  [unwired: 1 out]
        n588 = Build Array(w1889, w1888, w1887) -> (w1880:u32[])
        n589 = Split 1D Array(array=w1880, index="Number Interlace Sets") -> (first subarray=w1890:u32[])  [unwired: 1 out]
        n590 = Index Array(array=w1880, index=w1878) -> (element=w1879:u32)
        n591 = Add Array Elements(numeric array=w1890) -> (sum=w1884:u32)
        n592 = Select(t=w1884, s="Interlace", f=w1879) -> (s? t:f=→"Total Counts (ticks)":u32)
      }
      event "Reset Feedback": Value Change {
        n593 = event-data() -> ()  [unwired: 7 out]
        n594 = Unbundle By Name("Reset Feedback") -> ("Set 1"=w2035:bool, "Set 2"=w2034:bool)
        n595 = xnode "Read/Write Control"("FPGA VI Reference In"=w2037, "error in"=w2032, "FB Reset Set 1"=w2035, "FB Reset Set 2"=w2034) -> ("error out"=w2033:errorcluster)  [unwired: 1 out]
      }
      event "PID Gains": Value Change {
        n596 = event-data() -> ()  [unwired: 7 out]
        n597 = Unbundle By Name("PID Gains") -> ("Set 1"=w2100:T14, "Set 2"=w2099:T14)
        n598 = xnode "Read/Write Control"("FPGA VI Reference In"=w2101, "error in"=w2097, "FB Gains Set 1"=w2100, "FB Gains Set 2"=w2099) -> ("error out"=w2098:errorcluster)  [unwired: 1 out]
      }
      event "AI2 to Setpoint", "Trap Intensity\nSetpoints (V)": Value Change {
        n599 = event-data() -> ()  [unwired: 7 out]
        n600 = xnode "Read/Write Control"("FPGA VI Reference In"=w2176, "error in"=w2172) -> ("FPGA VI Reference Out"=w2175:T19, "error out"=w2174:errorcluster, "AI2 Y Sum Set 1"=w2183:i16, "AI2 Y Sum Set 2"=w2182:i16)
        n601 = Cluster To Array(cluster="AI2 to Setpoint") -> (array=w2186:bool[])
        n602 = local read "AI2 (V)"() -> (w2184:cluster{"Set 1":dbl, "Set 2":dbl})
        n603 = Or Array Elements(Boolean array=w2186) -> (logical OR=w2187:bool)
        n604 = Bundle By Name(cluster=w2184, "Set 1"=w2183, "Set 2"=w2182) -> (w2181:cluster{"Set 1":dbl, "Set 2":dbl})
        n605 = Divide(x=w2181, y=3276.7) -> (x/y=w2180:cluster{"Set 1":dbl, "Set 2":dbl})
        "AI2 (V)" <- w2180
        n606 = case shown="True" w2187 {
          tunnel: [w2251 w2268] -> w2179
          tunnel: "AI2 to Setpoint" -> [_ w2264]
          tunnel: "Trap Intensity\nSetpoints (V)" -> [w2252 w2267]
          tunnel: w2180 -> [_ w2261]
          frame False {
            n607 = Multiply(x=3276.7, y=w2252) -> (x*y=w2253:cluster{"Set 1":dbl, "Set 2":dbl})
            n608 = To Word Integer(number=w2253) -> (16bit integer=w2251:cluster{"Set 1":i16, "Set 2":i16})
          }
          frame True {
            n609 = Unbundle By Name(w2261) -> ("Set 1"=w2260:dbl, "Set 2"=w2259:dbl)
            n610 = Unbundle By Name(w2267) -> ("Set 1"=w2266:dbl, "Set 2"=w2265:dbl)
            n611 = Unbundle By Name(w2264) -> ("Set 1"=w2263:bool, "Set 2"=w2262:bool)
            n612 = Select(t=w2260, s=w2263, f=w2266) -> (s? t:f=w2258:dbl)
            n613 = Select(t=w2259, s=w2262, f=w2265) -> (s? t:f=w2257:dbl)
            n614 = Bundle By Name(cluster=w2267, "Set 1"=w2258, "Set 2"=w2257) -> (w2255:cluster{"Set 1":dbl, "Set 2":dbl})
            n615 = local write "Trap Intensity\nSetpoints (V)"(w2255) -> ()
            n616 = Multiply(x=3276.7, y=w2255) -> (x*y=w2256:cluster{"Set 1":dbl, "Set 2":dbl})
            n617 = To Word Integer(number=w2256) -> (16bit integer=w2268:cluster{"Set 1":i16, "Set 2":i16})
          }
        }
        n618 = Unbundle By Name(w2179) -> ("Set 1"=w2178:i16, "Set 2"=w2177:i16)
        n619 = xnode "Read/Write Control"("FPGA VI Reference In"=w2175, "error in"=w2174, "FB Setpoint Set 1"=w2178, "FB Setpoint Set 2"=w2177) -> ("error out"=w2173:errorcluster)  [unwired: 1 out]
      }
      event "Invert GI": Value Change {
        n620 = event-data() -> ()  [unwired: 7 out]
        n621 = xnode "Read/Write Control"("FPGA VI Reference In"=w2330, "error in"=w2328, "Invert GI"="Invert GI", "Invert GI 2"="Invert GI") -> ("error out"=w2329:errorcluster)  [unwired: 1 out]
      }
      event "Green FB Setpoint (mV)", "Green FB Gains", "Green FB On/Off", "Current When FB OFF (%)", "Green int current ON count adj": Value Change {
        n622 = event-data() -> ()  [unwired: 7 out]
        n623 = local read "Green FB Setpoint (mV)"() -> (w2396:dbl)
        n624 = local read "Current When FB OFF (%)"() -> (w2399:dbl)
        n625 = Multiply(x=w2396, y=3.2767) -> (x*y=w2395:dbl)
        n626 = Multiply(x=w2399, y=655.35) -> (x*y=w2400:dbl)
        n627 = To Unsigned Word Integer(number=w2400) -> (unsigned 16bit integer=w2398:u16)
        n628 = local read "Green int current ON count adj"() -> (w2403:u32)
        n629 = local read "Green FB Gains"() -> (w2402:T14)
        n630 = local read "Green Laser ON/Interlacing"() -> (w2393:bool)
        n631 = local read "Green laser mode"() -> (w2392:enum32{"Laser ON", "Laser OFF", "Interlace"})
        n632 = local read "Green FB On/Off"() -> (w2404:bool)
        n633 = Equal?(x=w2392, y=enum32{"Laser ON", "Laser OFF", "Interlace"}."Interlace") -> (x = y?=w2390:bool)
        n634 = Compound Arithmetic op=AND(w2390, w2404, w2393) -> (w2394:bool)
        n635 = xnode "Read/Write Control"("FPGA VI Reference In"=w2407, "error in"=w2406, "Green FB Setpoint"=w2395, "Green FB On/Off"=w2394, "Current Out"=w2398, "Green int current ON count adj"=w2403, "Green FB Gains"=w2402) -> ("error out"=w2405:errorcluster)  [unwired: 1 out]
      }
      event "Green laser mode", "Green Laser ON/Interlacing": Value Change {
        n636 = event-data() -> ()  [unwired: 7 out]
        n637 = case shown="True" "Green Laser ON/Interlacing" {
          tunnel: "Green laser mode" -> [_ w2545]
          tunnel: [enum32{"Laser ON", "Laser OFF", "Interlace"}."Laser OFF" ("Green laser mode") w2545] -> w2533
          tunnel: [FALSE w2541] -> w2532
          frame False {
          }
          frame True {
            n638 = local read "Green FB On/Off"() -> (w2542:bool)
            n639 = Equal?(x=w2545, y=enum32{"Laser ON", "Laser OFF", "Interlace"}."Interlace") -> (x = y?=w2543:bool)
            n640 = And(x=w2543, y=w2542) -> (x .and. y?=w2541:bool)
          }
        }
        n641 = xnode "Read/Write Control"("FPGA VI Reference In"=w2538, "error in"=w2536, "Operating Mode"=w2533, "Operating Mode 2"=w2533, "Green FB On/Off"=w2532) -> ("error out"=w2537:errorcluster)  [unwired: 1 out]
      }
      event "- phase (APD 1 Gate)", "+ phase (APD 1 Gate)": Value Change {
        n642 = event-data() -> ()  [unwired: 7 out]
        n643 = local read "Phase Adj. (APD 1 Gate)"() -> (w2624:i16)
        n644 = Negate(x=w2624) -> (-x=w2632:i16)
        n645 = Select(t=w2632, s="- phase (APD 1 Gate)", f=w2624) -> (s? t:f=w2631:i16)
        n646 = Or(x="- phase (APD 1 Gate)", y="+ phase (APD 1 Gate)") -> (x .or. y?=w2627:bool)
        n647 = xnode "Read/Write Control"("FPGA VI Reference In"=w2634, "error in"=w2633, "Phase count adjustment (APD 1 Gate)"=w2631) -> ("FPGA VI Reference Out"=w2629:T19, "error out"=w2630:errorcluster)
        n648 = xnode "Read/Write Control"("FPGA VI Reference In"=w2629, "error in"=w2630, "+ phase (APD 1 Gate)"=w2627) -> ("error out"=w2628:errorcluster)  [unwired: 1 out]
      }
      event "+ phase (APD 2 Gate)", "- phase (APD 2 Gate)": Value Change {
        n649 = event-data() -> ()  [unwired: 7 out]
        n650 = local read "Phase Adj. (APD 2 Gate)"() -> (w2710:i16)
        n651 = Negate(x=w2710) -> (-x=w2718:i16)
        n652 = Select(t=w2718, s="- phase (APD 2 Gate)", f=w2710) -> (s? t:f=w2717:i16)
        n653 = Or(x="- phase (APD 2 Gate)", y="+ phase (APD 2 Gate)") -> (x .or. y?=w2713:bool)
        n654 = xnode "Read/Write Control"("FPGA VI Reference In"=w2720, "error in"=w2719, "Phase count adjustment (APD 2 Gate)"=w2717) -> ("FPGA VI Reference Out"=w2715:T19, "error out"=w2716:errorcluster)
        n655 = xnode "Read/Write Control"("FPGA VI Reference In"=w2715, "error in"=w2716, "+ phase (APD 2 Gate)"=w2713) -> ("error out"=w2714:errorcluster)  [unwired: 1 out]
      }
      event "Phase Adj. (APD Acq)", "+ phase (APD Acq)", "- phase (APD Acq)": Value Change {
        n656 = event-data() -> ()  [unwired: 7 out]
        n657 = local read "Phase Adj. (APD Acq)"() -> (w2798:i16)
        n658 = Negate(x=w2798) -> (-x=w2804:i16)
        n659 = Select(t=w2804, s="+ phase (APD Acq)", f=w2798) -> (s? t:f=w2803:i16)
        n660 = Or(x="+ phase (APD Acq)", y="- phase (APD Acq)") -> (x .or. y?=w2799:bool)
        n661 = xnode "Read/Write Control"("FPGA VI Reference In"=w2806, "error in"=w2805, "Phase Count Adjustment (APD Acq)"=w2803) -> ("FPGA VI Reference Out"=w2801:T19, "error out"=w2802:errorcluster)
        n662 = xnode "Read/Write Control"("FPGA VI Reference In"=w2801, "error in"=w2802, "+ phase (APD Acq)"=w2799) -> ("error out"=w2800:errorcluster)  [unwired: 1 out]
      }
      event "Phase adj. (GI)", "+ phase (GI)", "- phase (GI)": Value Change {
        n663 = event-data() -> ()  [unwired: 7 out]
        n664 = Negate(x="Phase adj. (GI)") -> (-x=w2890:i16)
        n665 = Select(t=w2890, s="+ phase (GI)", f="Phase adj. (GI)") -> (s? t:f=w2889:i16)
        n666 = Or(x="+ phase (GI)", y="- phase (GI)") -> (x .or. y?=w2885:bool)
        n667 = xnode "Read/Write Control"("FPGA VI Reference In"=w2892, "error in"=w2891, "Phase count adjustment (GI)"=w2889) -> ("FPGA VI Reference Out"=w2887:T19, "error out"=w2888:errorcluster)
        n668 = xnode "Read/Write Control"("FPGA VI Reference In"=w2887, "error in"=w2888, "+ phase (GI)"=w2885) -> ("error out"=w2886:errorcluster)  [unwired: 1 out]
      }
      event "Phase adj. (GI) 2", "+ phase (GI) 2", "- phase (GI) 2": Value Change {
        n669 = event-data() -> ()  [unwired: 7 out]
        n670 = Negate(x="Phase adj. (GI) 2") -> (-x=w2976:i16)
        n671 = Select(t=w2976, s="+ phase (GI) 2", f="Phase adj. (GI) 2") -> (s? t:f=w2975:i16)
        n672 = Or(x="+ phase (GI) 2", y="- phase (GI) 2") -> (x .or. y?=w2971:bool)
        n673 = xnode "Read/Write Control"("FPGA VI Reference In"=w2978, "error in"=w2977, "Phase count adjustment (GI) 2"=w2975) -> ("FPGA VI Reference Out"=w2973:T19, "error out"=w2974:errorcluster)
        n674 = xnode "Read/Write Control"("FPGA VI Reference In"=w2973, "error in"=w2974, "+ phase (GI) 2"=w2971) -> ("error out"=w2972:errorcluster)  [unwired: 1 out]
      }
      event "Phase adj. (Green FB)", "- phase (Green FB)", "+ phase (Green FB)": Value Change {
        n675 = event-data() -> ()  [unwired: 7 out]
        n676 = Negate(x="Phase adj. (Green FB)") -> (-x=w3062:i16)
        n677 = Select(t=w3062, s="+ phase (Green FB)", f="Phase adj. (Green FB)") -> (s? t:f=w3061:i16)
        n678 = Or(x="+ phase (Green FB)", y="- phase (Green FB)") -> (x .or. y?=w3057:bool)
        n679 = xnode "Read/Write Control"("FPGA VI Reference In"=w3064, "error in"=w3063, "Phase count adjustment (Green FB)"=w3061) -> ("FPGA VI Reference Out"=w3059:T19, "error out"=w3060:errorcluster)
        n680 = xnode "Read/Write Control"("FPGA VI Reference In"=w3059, "error in"=w3060, "+ phase (Green FB)"=w3057) -> ("error out"=w3058:errorcluster)  [unwired: 1 out]
      }
      event "Invert APD Gate", "APD Gate ON Count", "APD Gate OFF Count", "APD Gate", "APD Integration Time (s)", "APD 1 AO Mult.", "APD 2 AO Mult.": Value Change {
        n681 = event-data() -> ()  [unwired: 7 out]
        n682 = local read "APD Integration Time (s)"() -> (w3140:dbl)
        n683 = local read "APD Gate ON Count"() -> (w3153:u32)
        n684 = local read "APD Gate OFF Count"() -> (w3152:u32)
        n685 = local read "Invert APD Gate"() -> (w3154:bool)
        n686 = local read "APD Gate"() -> (w3151:enum32{"ON", "OFF", "Interlace"})
        n687 = Multiply(x=w3140, y=40000000.0) -> (x*y=w3149:dbl)
        n688 = Reciprocal(x=w3140) -> (1/x=→"APD Acq Rate (Hz)":dbl)
        n689 = To Unsigned Long Integer(number=w3149) -> (unsigned 32bit integer=w3148:u32)
        n690 = local read "DMA Update Period (s)"() -> (w3141:dbl)
        n691 = Divide(x=w3141, y=w3140) -> (x/y=w3144:dbl)
        n692 = local read "APD 1 AO Mult."() -> (w3146:i16)
        n693 = local read "APD 2 AO Mult."() -> (w3145:i16)
        n694 = Multiply(x=2.0, y=w3144) -> (x*y=w3143:dbl)
        n695 = local write "APD Samples/FIFO Acq."(w3144) -> ()
        n696 = local write "APD Elements/DMA read"(w3143) -> ()